vi "HFRR ADV v038.vi"() -> ()   [LabVIEW 2025] (continued)
                }
                n3063 = control-ref of="Tab Control 9"() -> (w3828:refnum<vi>)
                n3064 = call-dynamic "Append Control Image to Report.vi"("report in"=w3833, "alignment (default)"=HTML_Report_Image_Alignment."ABSMIDDLE", "ctrl reference"=w3828, "error in (no error)"=w3832) -> ("report out"=w3827:refnum<class "NI_report.lvclass">, "error out"=w3826:errorcluster)  [unwired: 8 in, 2 out]
                n3065 = for {
                  N: 3 -> [_]
                  tunnel: [w3860] -> w3811
                  tunnel: [w3859] -> w3810
                  tunnel: w3827 -> [w3858]
                  tunnel: w3826 -> [w3857]
                  n3066 = call-dynamic "New Report Line.vi"("report in"=w3858, "error in (no error)"=w3857) -> ("report out"=w3860:refnum<class "NI_report.lvclass">, "error out"=w3859:errorcluster)  [unwired: 12 in]
                }
                n3067 = for {
                  N: 100 -> [_]
                  tunnel: w3811 -> [w3856]
                  tunnel: w3810 -> [w3854]
                  tunnel: [w3855] -> w3807
                  tunnel: [w3853] -> w3805
                  n3068 = call-dynamic "Set Report Tab Width.vi"("report in"=w3856, "error in (no error)"=w3854) -> ("report out"=w3855:refnum<class "NI_report.lvclass">, "error out"=w3853:errorcluster)  [unwired: 12 in]
                }
                n3069 = String To Path(string="C:\\LAB-IQ\\im\\Temp_resized.jpg") -> (path=w3797:path)
                n3070 = call-poly <vilib>:"Append Image to Report.vi"("report in"=w3807, "path or URL of image"=w3797, "error in (no error)"=w3805) -> ("report out"=w3806:refnum<class "NI_report.lvclass">, "error out"=w3804:errorcluster)  [unwired: 9 in, 2 out]
                n3071 = call-poly <vilib>:"Open HTML Report in Browser.vi"("report in"=w3806, "error in (no error)"=w3804) -> ("report out"=w3841:refnum<class "NI_report.lvclass">, "error out"=w3840:errorcluster)  [unwired: 11 in, 1 out]
                n3072 = call-dynamic "Dispose Report.vi"("report in"=w3841, "error in (no error)"=w3840) -> ()  [unwired: 13 in, 1 out]
              }
              frame #2 {
              }
              frame #3 {
                n3073 = disable-structure shown="Disabled" {
                  frame Disabled {
                    n3074 = local read "String 10"() -> (w3881:string)
                    n3075 = Concatenate Strings("C:\\LAB-IQ-NXT\\Data\\" ("string"), w3881, ".jpg" ("string")) -> (w3879:string)
                    n3076 = String To Path(string=w3879) -> (path=w3878:path)
                    n3077 = Delete(path (use dialog)=w3878) -> ()  [unwired: 4 in, 3 out]
                  }
                  frame Enabled {
                  }
                }
                n3078 = local write "Print 2"(FALSE ("Print")) -> ()
              }
            }
          }
        }
      }
    }
    n3079 = Wait (ms)(milliseconds to wait=u32 50) -> ()  [unwired: 1 out]
    n3080 = Wait (ms)(milliseconds to wait=u32 50) -> ()  [unwired: 1 out]
    n3081 = local read "Quit"() -> (w2223:bool)
  }
  n3082 = VISA Close(VISA resource name=w41, error in (no error)=w40) -> ()  [unwired: 1 out]
  n3083 = while {
    stop <- w4032 stop-if-true
    n3084 = local read "Auto Start Test"() -> (w4030:bool)
    n3085 = local read "RUN"() -> (w4029:bool)
    n3086 = Wait (ms)(milliseconds to wait=u32 1000) -> ()  [unwired: 1 out]
    n3087 = Or(x=w4029, y=w4030) -> (x .or. y?=w4028:bool)
    n3088 = case shown="True" w4028 {
      frame False {
      }
      frame True {
        n3089 = local read "LVDT STROKE Actual"() -> (w4033:dbl)
        n3090 = In Range and Coerce(upper limit=1.2, x=w4033, lower limit=0.6) -> (In Range?=w4036:bool)  [unwired: 1 out]
        n3091 = call-poly <vilib>:"Random Number (Range).vi"("lower bound (0)"=0.998 ("upper bound (100)"), "upper bound (100)"=1.003) -> ("number"=w4034:dbl)  [unwired: 9 in]
        n3092 = case shown="True" w4036 {
          tunnel: [w4041 w4042] -> w4035
          tunnel: w4034 -> [_ w4042]
          tunnel: w4033 -> [w4041 _]
          frame False {
          }
          frame True {
          }
        }
        "LVDT STROKE DISPLAY" <- w4035
      }
    }
    n3093 = local read "Quit"() -> (w4032:bool)
  }
  n3094 = while {
    tunnel: [w4059] -> w49
    shift-right: [w4052] -> _
    shift-left: 0.0 -> [w4055]
    shift-right: [w4051] -> _
    shift-left: 0.0 -> [w4054]
    shift-right: [w4050] -> _
    shift-left: 100.0 ("vc_cmd") -> [w4053]
    stop <- w4059 stop-if-true
    # "PID LOGIC"
    n3095 = local read "run test Calibration"() -> (w4047:bool)
    n3096 = local read "RUN"() -> (w4057:bool)
    n3097 = local read "Auto Start Temp"() -> (w4048:bool)
    n3098 = local read "Auto Start Test"() -> (w4056:bool)
    n3099 = local read "START TEMP"() -> (w4046:bool)
    n3100 = And(x=w4048, y=w4056) -> (x .and. y?=w4049:bool)
    n3101 = Or(x=w4057, y=w4049) -> (x .or. y?=w4058:bool)
    n3102 = And(x=w4058, y=w4046) -> (x .and. y?=w4045:bool)
    n3103 = And(x=w4047, y=w4046) -> (x .and. y?=w4044:bool)
    n3104 = Or(x=w4044, y=w4045) -> (x .or. y?=w4043:bool)
    n3105 = Wait (ms)(milliseconds to wait="milliseconds to wait") -> ()  [unwired: 1 out]
    n3106 = case shown="True" w4043 {
      tunnel: [400.0 ("out_vc_cmd") w4078] -> w4050
      tunnel: [w4062 w4080] -> w4051
      tunnel: [w4062 w4079] -> w4052
      tunnel: w4055 -> [_ w4069]
      tunnel: w4054 -> [_ w4068]
      tunnel: w4053 -> [_ w4067]
      tunnel: w4047 -> [_ w4063]
      frame False {
        w4062 = 0.0 ("error_out")
      }
      frame True {
        n3107 = case shown="True" w4063 {
          tunnel: [w4087 1.0] -> w4065
          frame False {
            n3108 = local read "Set Strk"() -> (w4086:dbl)
            n3109 = Add(x=w4086, y="Add up Stroke") -> (x+y=w4087:dbl)
          }
          frame True {
          }
        }
        n3110 = local read "LVDT STROKE"() -> (w4064:dbl)
        n3111 = formula code="// Zero-Hardcode Explicit Positional-Form PID Engine\n// Inputs: target_stroke, measured_stroke, dt, prev_error, integral_accumulator_in, prev_vc_cmd\n//         kp, ki, kd, max_step_change, max_amplitude, min_amplitude, startup_cmd\n// Outputs: vc_cmd, error_out, out_error, integral_accumulator_out, out_vc_cmd\n\n// 1. Calculate Tracking Error\nfloat current_error = target_stroke - measured_stroke;\nerror_out = current_error;\n\n// 2. Compute Proportional Term\nfloat p_term = kp * current_error;\n\n// 3. Compute Derivative Term\nfloat d_term = 0.0;\nif (dt > 0.0) {\n    d_term = kd * ((current_error - prev_error) / dt);\n}\n\n// 4. Update and Accumulate Integral Term\nfloat current_integral = integral_accumulator_in + (current_error * dt);\nfloat i_term = ki * current_integral;\n\n// 5. Calculate Ideal Target Command (Anchored by startup baseline)\nfloat ideal_command = startup_cmd + p_term + i_term + d_term;\n\n// 6. Apply Loop Rate Limiting FIRST \n// (Forces the command to climb gradually from prev_vc_cmd instead of jumping straight to max)\nfloat raw_adjustment = ideal_command - prev_vc_cmd;\n\nif (raw_adjustment > max_step_change) {\n    raw_adjustment = max_step_change;\n} else if (raw_adjustment < -max_step_change) {\n    raw_adjustment = -max_step_change;\n}\n\nfloat next_vc_cmd = prev_vc_cmd + raw_adjustment;\n\n// 7. Anti-Windup Protection & Final Output Safety Safeguard Clamping\n// (Back-calculating based on what we are ACTUALLY outputting)\nif (next_vc_cmd > max_amplitude) {\n    float excess = next_vc_cmd - max_amplitude;\n    if (ki > 0.0) {\n        current_integral -= excess / ki;\n    }\n    next_vc_cmd = max_amplitude;\n} else if (next_vc_cmd < min_amplitude) {\n    float excess = next_vc_cmd - min_amplitude;\n    if (ki > 0.0) {\n        current_integral -= excess / ki;\n    }\n    next_vc_cmd = min_amplitude;\n}\n\n// 8. Map to Shift Registers for memory persistence\nvc_cmd = next_vc_cmd;\nout_error = current_error;                   \nintegral_accumulator_out = current_integral;  \nout_vc_cmd = next_vc_cmd;"("target_stroke"=w4065, "measured_stroke"=w4064, "dt"="dt", "integral_accumulator_in"=w4068, "prev_error"=w4069, "prev_vc_cmd"=w4067, "kp"="kp", "ki"="ki", "kd"="kd", "max_step_change"="max_step_change", "max_amplitude"="max_amplitude", "min_amplitude"="min_amplitude", "startup_cmd"="startup_cmd") -> ("vc_cmd"=w4084:dbl, "out_error"=w4079:dbl, "integral_accumulator_out"=w4080:dbl, "out_vc_cmd"=w4078:dbl)  [unwired: 1 out]
        "output Vpp" <- w4084
        n3112 = Number To Fractional String(number=w4084, precision (6)=i16 1) -> (F-format string=w4082:string)  [unwired: 2 in]
        n3113 = Concatenate Strings("DAC;" ("string"), w4082) -> (w4066:string)
        n3114 = local write "Due Write"(w4066) -> ()
        "prev_error" <- w4069
        "integral_accumulator_in" <- w4068
        "prev_vc_cmd" <- w4067
      }
    }
    n3115 = local read "Quit"() -> (w4059:bool)
  }
  n3116 = Or(x=w45, y=w44) -> (x .or. y?=w46:bool)
  n3117 = Or(x=w42, y=w46) -> (x .or. y?=w51:bool)
  n3118 = control-ref of="new picture"() -> ()  [unwired: 1 out]
  n3119 = Or(x=w54, y=w51) -> (x .or. y?=w48:bool)
  n3120 = Or(x=w48, y=w49) -> (x .or. y?=w43:bool)
  n3121 = while {
    tunnel: [w4089] -> w53
    i -> [w4096]
    stop <- w4089 stop-if-true
    n3122 = local read "Quit"() -> (w4089:bool)
    n3123 = Equal To 0?(x=w4096) -> (x = 0?=w4094:bool)
    n3124 = call "Elapsed Time3"("Time Target (s)"=45.0, "Auto Reset"=TRUE) -> ("Time has Elapsed"=w4093:bool)  [unwired: 10 in, 7 out]
    n3125 = Wait (ms)(milliseconds to wait=u32 50) -> ()  [unwired: 1 out]
    n3126 = Or(x=w4093, y=w4094) -> (x .or. y?=w4095:bool)
    n3127 = case shown="True" w4095 {
      frame False {
      }
      frame True {
        n3128 = call <vilib>:"System Exec.vi"("run minimized? (F)"=TRUE, "error in (no error)"="error in (no error)", "command line"="powercfg.exe -change -monitor-timeout-ac 0") -> ("error out"=w4107:errorcluster)  [unwired: 5 in, 3 out]
        n3129 = call <vilib>:"System Exec.vi"("run minimized? (F)"=TRUE, "error in (no error)"=w4107, "command line"="powercfg.exe -change -disk-timeout-ac 0") -> ("error out"=w4106:errorcluster)  [unwired: 5 in, 3 out]
        n3130 = call <vilib>:"System Exec.vi"("run minimized? (F)"=TRUE, "error in (no error)"=w4106, "command line"="powercfg.exe -change -standby-timeout-ac 0") -> ("error out"=w4105:errorcluster)  [unwired: 5 in, 3 out]
        n3131 = call <vilib>:"System Exec.vi"("run minimized? (F)"=TRUE, "error in (no error)"=w4105, "command line"="powercfg.exe -change -hibernate-timeout-ac 0") -> ("error out"=w4104:errorcluster)  [unwired: 5 in, 3 out]
        n3132 = call <vilib>:"Simple Error Handler.vi"("error in (no error)"=w4104) -> ("error out"=w4110:errorcluster)  [unwired: 4 in, 4 out]
        n3133 = call <vilib>:"Clear Errors.vi"("error in (no error)"=w4110) -> ("error out"=→"error out":errorcluster)  [unwired: 5 in, 1 out]
      }
    }
  }
  n3134 = Compound Arithmetic op=OR(w56, w43, w53) -> (w55:bool)
  n3135 = flat-sequence {
    tunnel: w55 -> [_]
    tunnel: [w4112] -> w25
    tunnel: w25 -> [_]
    frame #0 {
      n3136 = call "CLOSE CONNECTION.vi"() -> ("error out"=w4112:errorcluster)  [unwired: 11 in]
    }
    frame #1 {
      n3137 = Quit LabVIEW(quit? (T)=TRUE) -> ()
      n3138 = local write "Quit"(FALSE ("EXIT")) -> ()
    }
  }
  n3139 = property on="Heater Button" class="Bool (strict)"("Visible"=TRUE) -> ()  [unwired: 2 in, 2 out]
  n3140 = while {
    tunnel: [w4119] -> _
    i -> [w4119]
    stop <- w4115 stop-if-true
    # "Langauage selection"
    n3141 = Equal?(x="Lan flag", y=22.0) -> ()  [unwired: 1 out]
    n3142 = disable-structure shown="Disabled" {
      frame Disabled {
        n3143 = stacked-sequence {
          frame #0 {
            n3144 = case shown="\"Russian\"" "Language Selection" {
              tunnel: [0 1] -> w4121
              frame "English", Default {
              }
              frame "Russian" {
              }
            }
            n3145 = for {
              N: 130 -> [_]
              tunnel: "Table" -> [w4130]
              tunnel: w4121 -> [w4129]
              i -> [w4128]
              n3146 = Index Array(array=w4130, index (row)=w4128, index (col)=w4129) -> (element=w4127:string)
              n3147 = case shown="1" w4128 {
                tunnel: w4127 -> [w4131 w4132 _ w4133 w4134 w4135 w4136 w4137 w4138 w4139 w4140 w4141 w4142 w4143 w4144 w4145 w4146 w4147 w4148 w4149 w4150 w4151 w4152 w4153 w4154 w4155 w4156 w4157 w4158 _ _ w4159 w4160 w4161 w4162 w4163 w4164 w4173 w4180 w4187 w4194 w4198 w4201 w4204 w4206 w4208 w4209 w4210 w4211 w4212 w4213 w4214 w4215 w4216 w4217 w4218 w4219 w4220 w4221 w4222 w4223 w4224 w4225 w4226 w4227 w4228 w4229 w4230 w4231 w4232 w4233 w4234 w4235 w4236 w4237 w4238 w4239 w4240 w4241 w4242 w4243 w4244 w4245 w4246 w4247 w4248 w4249 w4250 w4251 w4252 w4253 w4254 w4255 w4256 w4257 w4258 w4259 w4260 w4261 w4262 w4263 w4264 w4265 w4266 w4267 _ w4268 w4269 w4270 w4271 w4272 w4273 w4274 w4275 w4276 w4277 w4278 w4279 w4280 _ w4281 w4282 w4283 w4284 w4285 w4286 _]
                frame 0 {
                  n3148 = local write "S"(w4131) -> ()
                }
                frame 1 {
                  n3149 = local write "S 2"(w4132) -> ()
                }
                frame 2 {
                }
                frame 3 {
                  n3150 = local write "S 4"(w4133) -> ()
                }
                frame 4 {
                  n3151 = property on="FILE" class="Str"("Caption.Text"=w4134) -> ()  [unwired: 2 in, 2 out]
                }
                frame 5 {
                  n3152 = property on="Fuel Discription :" class="Str"("Caption.Text"=w4135) -> ()  [unwired: 2 in, 2 out]
                }
                frame 6 {
                  n3153 = property on="Remarks :" class="Str"("Caption.Text"=w4136) -> ()  [unwired: 2 in, 2 out]
                }
                frame 7 {
                  n3154 = property on="Save & Continue" class="Bool (strict)"("Boolean Text.Text"=w4137) -> ()  [unwired: 2 in, 2 out]
                }
                frame 8 {
                }
                frame 9 {
                  n3155 = property on="Set Hz" class="DigNum (strict)"("Caption.Text"=w4139) -> ()  [unwired: 2 in, 2 out]
                }
                frame 10 {
                }
                frame 11 {
                  n3156 = property on="NORMAL LOAD" class="DigNum (strict)"("Caption.Text"=w4141) -> ()  [unwired: 2 in, 2 out]
                }
                frame 12 {
                }
                frame 13 {
                  n3157 = property on="Set Temp" class="DigNum (strict)"("Caption.Text"=w4143) -> ()  [unwired: 2 in, 2 out]
                }
                frame 14 {
                  n3158 = local write "S 15"(w4144) -> ()
                }
                frame 15 {
                  n3159 = property on="Set Rh" class="DigNum (strict)"("Caption.Text"=w4145) -> ()  [unwired: 2 in, 2 out]
                }
                frame 16 {
                }
                frame 17 {
                  n3160 = local write "S 18"(w4147) -> ()
                }
                frame 18 {
                  "String 17" <- w4148
                }
                frame 19 {
                  n3161 = property on="test time" class="DigNum (strict)"("Caption.Text"=w4149) -> ()  [unwired: 2 in, 2 out]
                }
                frame 20 {
                  "String 18" <- w4150
                  "String 22" <- w4150
                }
                frame 21 {
                  n3162 = property on="Elapsed time" class="DigNum (strict)"("Caption.Text"=w4151) -> ()  [unwired: 2 in, 2 out]
                }
                frame 22 {
                  n3163 = property on="Samplingtime 2" class="DigNum (strict)"("Caption.Text"=w4152) -> ()  [unwired: 2 in, 2 out]
                }
                frame 23 {
                  "String 21" <- w4153
                }
                frame 24 {
                  n3164 = property on="Countdown" class="DigNum (strict)"("Caption.Text"=w4154) -> ()  [unwired: 2 in, 2 out]
                }
                frame 25 {
                  n3165 = property on="Countdown 2" class="DigNum (strict)"("Caption.Text"=w4155) -> ()  [unwired: 2 in, 2 out]
                }
                frame 26 {
                  n3166 = property on="Engage" class="Bool (strict)"("Boolean Text.Text"=w4156) -> ()  [unwired: 2 in, 2 out]
                }
                frame 27 {
                  n3167 = property on="Boolean  4" class="Bool (strict)"("Boolean Text.Text"=w4157) -> ()  [unwired: 2 in, 2 out]
                }
                frame 28 {
                  n3168 = property on="Test \nStatus" class="Bool (strict)"("Boolean Text.Text"=w4158) -> ()  [unwired: 2 in, 2 out]
                }
                frame 29 {
                }
                frame 30 {
                }
                frame 31 {
                }
                frame 32 {
                  n3169 = property on="RSTCOF" class="Bool"("Boolean Text.Text"=w4160) -> ()  [unwired: 2 in, 2 out]
                  n3170 = property on="RST FF" class="Bool"("Boolean Text.Text"=w4160) -> ()  [unwired: 2 in, 2 out]
                  n3171 = property on="RST TEMP" class="Bool"("Boolean Text.Text"=w4160) -> ()  [unwired: 2 in, 2 out]
                  n3172 = property on="RSTV1 3" class="Bool"("Boolean Text.Text"=w4160) -> ()  [unwired: 2 in, 2 out]
                  n3173 = property on="rstv2" class="Bool"("Boolean Text.Text"=w4160) -> ()  [unwired: 2 in, 2 out]
                  n3174 = property on="RSTV1 2" class="Bool"("Boolean Text.Text"=w4160) -> ()  [unwired: 2 in, 2 out]
                  n3175 = property on="RST CP" class="Bool"("Boolean Text.Text"=w4160) -> ()  [unwired: 2 in, 2 out]
                }
                frame 33 {
                  "S 61" <- w4161
                }
                frame 34 {
                  "String 23" <- w4162
                }
                frame 35 {
                  n3176 = property on="Rh Before" class="DigNum (strict)"("Caption.Text"=w4163) -> ()  [unwired: 2 in, 2 out]
                }
                frame 36 {
                  n3177 = Match Pattern(string=w4164, regular expression=",") -> (before substring=→"bs":string, after substring=→"as":string)  [unwired: 1 in, 2 out]
                  n3178 = property on="Rh After" class="DigNum (strict)"("Caption.Text"=w4164) -> ()  [unwired: 2 in, 2 out]
                }
                frame 37 {
                  n3179 = Match Pattern(string=w4173, regular expression=",") -> (before substring=w4172:string, after substring=w4171:string)  [unwired: 1 in, 2 out]
                  "bs" <- w4172
                  "as" <- w4171
                  n3180 = Concatenate Strings(w4172, w4171) -> (w4168:string)
                  n3181 = property on="Humidity before test 2" class="DigNum (strict)"("Caption.Text"=w4168) -> ()  [unwired: 2 in, 2 out]
                  n3182 = Concatenate Strings(w4168, "=" ("string")) -> (w4169:string)
                  n3183 = local write "S 38"(w4169) -> ()
                }
                frame 38 {
                  n3184 = Match Pattern(string=w4180, regular expression=",") -> (before substring=w4179:string, after substring=w4178:string)  [unwired: 1 in, 2 out]
                  "bs" <- w4179
                  "as" <- w4178
                  n3185 = Concatenate Strings(w4179, w4178) -> (w4175:string)
                  n3186 = property on="Humidity after test 2" class="DigNum (strict)"("Caption.Text"=w4175) -> ()  [unwired: 2 in, 2 out]
                  n3187 = Concatenate Strings(w4175, "=" ("string")) -> (w4177:string)
                  n3188 = local write "S 39"(w4177) -> ()
                }
                frame 39 {
                  n3189 = Match Pattern(string=w4187, regular expression=",") -> (before substring=w4186:string, after substring=w4185:string)  [unwired: 1 in, 2 out]
                  "bs" <- w4186
                  "as" <- w4185
                  n3190 = Concatenate Strings(w4186, w4185) -> (w4182:string)
                  n3191 = property on="Temperature before test 2" class="DigNum (strict)"("Caption.Text"=w4182) -> ()  [unwired: 2 in, 2 out]
                  n3192 = Concatenate Strings(w4182, "=" ("string")) -> (→"String 34":string)
                }
                frame 40 {
                  n3193 = Match Pattern(string=w4194, regular expression=",") -> (before substring=w4193:string, after substring=w4192:string)  [unwired: 1 in, 2 out]
                  "bs" <- w4193
                  "as" <- w4192
                  n3194 = Concatenate Strings(w4193, w4192) -> (w4189:string)
                  n3195 = property on="Temperature after test 2" class="DigNum (strict)"("Caption.Text"=w4189) -> ()  [unwired: 2 in, 2 out]
                  n3196 = Concatenate Strings(w4189, "=" ("string")) -> (→"String 35":string)
                  n3197 = property on="Temperature after test" class="DigNum (strict)"("Caption.Text"=w4189) -> ()  [unwired: 2 in, 2 out]
                }
                frame 41 {
                  n3198 = property on="AVP 2" class="DigNum (strict)"("Caption.Text"=w4198) -> ()  [unwired: 2 in, 2 out]
                  n3199 = Concatenate Strings(w4198, "=" ("string")) -> (→"String 36":string)
                }
                frame 42 {
                  n3200 = property on="MWSD 2" class="DigNum (strict)"("Caption.Text"=w4201) -> ()  [unwired: 2 in, 2 out]
                  n3201 = Concatenate Strings(w4201, "=" ("string")) -> (→"String 37":string)
                }
                frame 43 {
                  n3202 = property on="HCF 2" class="DigNum (strict)"("Caption.Text"=w4204) -> ()  [unwired: 2 in, 2 out]
                  n3203 = Concatenate Strings(w4204, "=" ("string")) -> (→"String 38":string)
                }
                frame 44 {
                  n3204 = Concatenate Strings(w4206, "=" ("string")) -> (→"String 39":string)
                  n3205 = property on="WS1.4 2" class="DigNum (strict)"("Caption.Text"=w4206) -> ()  [unwired: 2 in, 2 out]
                }
                frame 45 {
                }
                frame 46 {
                  n3206 = local write "S 47"(w4209) -> ()
                }
                frame 47 {
                  n3207 = local write "S 48"(w4210) -> ()
                }
                frame 48 {
                  n3208 = local write "S 49"(w4211) -> ()
                }
                frame 49 {
                  n3209 = local write "S 50"(w4212) -> ()
                }
                frame 50 {
                  n3210 = local write "S 51"(w4213) -> ()
                }
                frame 51 {
                  n3211 = local write "S 52"(w4214) -> ()
                }
                frame 52 {
                  n3212 = local write "S 53"(w4215) -> ()
                }
                frame 53 {
                  n3213 = local write "S 54"(w4216) -> ()
                }
                frame 54 {
                  n3214 = local write "S 55"(w4217) -> ()
                }
                frame 55 {
                  n3215 = local write "S 56"(w4218) -> ()
                }
                frame 56 {
                  n3216 = local write "S 57"(w4219) -> ()
                }
                frame 57 {
                  n3217 = local write "S 58"(w4220) -> ()
                }
                frame 58 {
                  n3218 = local write "S 59"(w4221) -> ()
                }
                frame 59 {
                  n3219 = local write "S 60"(w4222) -> ()
                }
                frame 60 {
                  n3220 = local write "S 62"(w4223) -> ()
                }
                frame 61 {
                  n3221 = local write "S 63"(w4224) -> ()
                }
                frame 62 {
                  n3222 = local write "S 64"(w4225) -> ()
                }
                frame 63 {
                  n3223 = local write "S 65"(w4226) -> ()
                }
                frame 64 {
                  n3224 = local write "S 66"(w4227) -> ()
                }
                frame 65 {
                  n3225 = local write "S 67"(w4228) -> ()
                }
                frame 66 {
                  n3226 = local write "S 68"(w4229) -> ()
                }
                frame 67 {
                  n3227 = local write "S 69"(w4230) -> ()
                }
                frame 68 {
                  n3228 = local write "S 70"(w4231) -> ()
                }
                frame 69 {
                  n3229 = local write "S 71"(w4232) -> ()
                }
                frame 70 {
                  n3230 = local write "S 72"(w4233) -> ()
                }
                frame 71 {
                  n3231 = local write "S 73"(w4234) -> ()
                }
                frame 72 {
                  n3232 = local write "S 74"(w4235) -> ()
                }
                frame 73 {
                  n3233 = local write "S 75"(w4236) -> ()
                }
                frame 74 {
                  n3234 = local write "S 76"(w4237) -> ()
                }
                frame 75 {
                  n3235 = local write "S 77"(w4238) -> ()
                }
                frame 76 {
                  n3236 = local write "S 78"(w4239) -> ()
                }
                frame 77 {
                  n3237 = local write "S 79"(w4240) -> ()
                }
                frame 79 {
                  n3238 = property on="Sample Temperature ( °C )" class="XYGraph (strict)"("Y Scale.Name Label.Text"=w4241) -> ()  [unwired: 2 in, 2 out]
                }
                frame 80 {
                  n3239 = local write "S 81"(w4242) -> ()
                  n3240 = property on="Humidity ( %RH )" class="XYGraph (strict)"("Y Scale.Name Label.Text"=w4242) -> ()  [unwired: 2 in, 2 out]
                }
                frame 78 {
                  n3241 = property on="Air Temperature  ( °C )" class="XYGraph (strict)"("X Scale.Name Label.Text"=w4243) -> ()  [unwired: 2 in, 2 out]
                  n3242 = property on="Humidity ( %RH )" class="XYGraph (strict)"("X Scale.Name Label.Text"=w4243) -> ()  [unwired: 2 in, 2 out]
                  n3243 = property on="Sample Temperature ( °C )" class="XYGraph (strict)"("X Scale.Name Label.Text"=w4243) -> ()  [unwired: 2 in, 2 out]
                  n3244 = property on="Coefficient Of Friction" class="XYGraph (strict)"("X Scale.Name Label.Text"=w4243) -> ()  [unwired: 2 in, 2 out]
                }
                frame 81 {
                  n3245 = property on="Air Temperature  ( °C )" class="XYGraph (strict)"("Y Scale.Name Label.Text"=w4244) -> ()  [unwired: 2 in, 2 out]
                }
                frame 82 {
                  n3246 = local write "S 84"(w4245) -> ()
                }
                frame 83 {
                  n3247 = local write "S 85"(w4246) -> ()
                }
                frame 84 {
                  n3248 = local write "S 86"(w4247) -> ()
                }
                frame 85 {
                  n3249 = local write "S 87"(w4248) -> ()
                }
                frame 86 {
                  n3250 = local write "S 88"(w4249) -> ()
                }
                frame 87 {
                }
                frame 88 {
                  n3251 = local write "S 90"(w4251) -> ()
                }
                frame 89 {
                  n3252 = local write "S 91"(w4252) -> ()
                }
                frame 90 {
                  n3253 = local write "S 92"(w4253) -> ()
                }
                frame 91 {
                  n3254 = local write "S 93"(w4254) -> ()
                }
                frame 92 {
                  n3255 = local write "S 94"(w4255) -> ()
                }
                frame 93 {
                  n3256 = local write "S 95"(w4256) -> ()
                }
                frame 94 {
                  n3257 = local write "S 96"(w4257) -> ()
                }
                frame 95 {
                  n3258 = local write "S 97"(w4258) -> ()
                }
                frame 96 {
                  n3259 = local write "S 98"(w4259) -> ()
                }
                frame 97 {
                  n3260 = local write "S 99"(w4260) -> ()
                }
                frame 98 {
                  n3261 = local write "S 100"(w4261) -> ()
                }
                frame 99 {
                  n3262 = local write "S 101"(w4262) -> ()
                }
                frame 100 {
                  n3263 = local write "S 102"(w4263) -> ()
                }
                frame 101 {
                  n3264 = local write "S 103"(w4264) -> ()
                }
                frame 102 {
                  n3265 = local write "S 104"(w4265) -> ()
                }
                frame 103 {
                  n3266 = local write "S 105"(w4266) -> ()
                }
                frame 104 {
                  n3267 = local write "S 106"(w4267) -> ()
                }
                frame 105 {
                }
                frame 106 {
                  n3268 = property on="OK Button 17" class="Bool (strict)"("Boolean Text.Text"=w4268) -> ()  [unwired: 2 in, 2 out]
                }
                frame 107 {
                  n3269 = property on="OK Button 16" class="Bool (strict)"("Boolean Text.Text"=w4269) -> ()  [unwired: 2 in, 2 out]
                }
                frame 108 {
                  n3270 = property on="TITTLE" class="Str"("Caption.Text"=w4270) -> ()  [unwired: 2 in, 2 out]
                }
                frame 109 {
                  "String 30" <- w4271
                }
                frame 110 {
                  n3271 = property on="Test Date" class="Str"("Caption.Text"=w4272) -> ()  [unwired: 2 in, 2 out]
                  "String 31" <- w4272
                }
                frame 111 {
                  n3272 = property on="Sample ID" class="Str"("Caption.Text"=w4273) -> ()  [unwired: 2 in, 2 out]
                  "String 32" <- w4273
                }
                frame 112 {
                  n3273 = property on="Tested by" class="Str"("Caption.Text"=w4274) -> ()  [unwired: 2 in, 2 out]
                  "String 33" <- w4274
                }
                frame 113 {
                  n3274 = property on="System Configured Printers 2" class="Arr (strict)"("Caption.Text"=w4275) -> ()  [unwired: 2 in, 2 out]
                }
                frame 114 {
                  n3275 = property on="Selected Printer" class="Str"("Caption.Text"=w4276) -> ()  [unwired: 2 in, 2 out]
                }
                frame 115 {
                  n3276 = property on="Select Printer 3" class="DigNum (strict)"("Caption.Text"=w4277) -> ()  [unwired: 2 in, 2 out]
                }
                frame 116 {
                  n3277 = property on="Print" class="Bool (strict)"("Boolean Text.Text"=w4278) -> ()  [unwired: 2 in, 2 out]
                }
                frame 117 {
                  "String 41" <- w4279
                }
                frame 118 {
                  n3278 = property on="tested by" class="Str"("Caption.Text"=w4280) -> ()  [unwired: 2 in, 2 out]
                }
                frame 119 {
                }
                frame 120 {
                  n3279 = property on="Export" class="Bool (strict)"("Boolean Text.Text"=w4281) -> ()  [unwired: 2 in, 2 out]
                }
                frame 121 {
                }
                frame 122 {
                }
                frame 123 {
                  n3280 = property on="Select File Type" class="Enum (strict)"("Caption.Text"=w4284) -> ()  [unwired: 2 in, 2 out]
                }
                frame 124 {
                  n3281 = property on="s.NO" class="Str"("Caption.Text"=w4285) -> ()  [unwired: 2 in, 2 out]
                  "String 45" <- w4285
                }
                frame 125 {
                  n3282 = property on="trip1 8" class="Bool (strict)"("Boolean Text.Text"=w4286) -> ()  [unwired: 2 in, 2 out]
                }
                frame 126, Default {
                }
              }
            }
          }
          frame #1 {
            w4294 = TRUE ("Visible")
            n3283 = local read "S 91"() -> (w4311:string)
            n3284 = local read "S 90"() -> (w4310:string)
            n3285 = local read "S 88"() -> (w4309:string)
            n3286 = property on="File Path" class="Path"("Caption.Text"=w4310) -> ()  [unwired: 2 in, 2 out]
            n3287 = local read "S 71"() -> (w4304:string)
            n3288 = local read "S 86"() -> (w4306:string)
            n3289 = local read "S 85"() -> (w4307:string)
            n3290 = local read "S 87"() -> (w4305:string)
            n3291 = local read "S 84"() -> (w4308:string)
            n3292 = local read "S 103"() -> (w4293:string)
            n3293 = local read "S 104"() -> (w4292:string)
            n3294 = property on="Password" class="Str"("Caption.Text"=w4307) -> ()  [unwired: 2 in, 2 out]
            n3295 = property on="EDIT" class="Bool (strict)"("Boolean Text.Text"=w4304) -> ()  [unwired: 2 in, 2 out]
            n3296 = property on="SAVE" class="Bool (strict)"("Boolean Text.Text"=w4308) -> ()  [unwired: 2 in, 2 out]
            n3297 = Build Array(w4293, w4292) -> (w4291:string[])
            n3298 = property on="Heater Button" class="Bool (strict)"("Strings [4]"=w4291) -> ()  [unwired: 2 in, 2 out]
            n3299 = local read "S 92"() -> (w4303:string)
            n3300 = local read "S 93"() -> (w4302:string)
            n3301 = local read "S 105"() -> (w4289:string)
            n3302 = local read "S 106"() -> (w4288:string)
            n3303 = Build Array(w4303, w4302) -> ()  [unwired: 1 out]
            n3304 = Build Array(w4289, w4288) -> (w4290:string[])
            n3305 = local read "S 95"() -> (w4300:string)
            n3306 = local read "S 94"() -> (w4301:string)
            n3307 = local read "bs"() -> (w4316:string)
            n3308 = local read "as"() -> (w4317:string)
            n3309 = property on="Humidity" class="Bool (strict)"("Strings [4]"=w4290) -> ()  [unwired: 2 in, 2 out]
            n3310 = Concatenate Strings(w4316, "\r", w4317) -> ()  [unwired: 1 out]
            n3311 = property on="Rh After" class="DigNum (strict)"("Caption.Size to Text?"=TRUE ("Caption.Size to Text")) -> ()  [unwired: 2 in, 2 out]
            n3312 = local read "S 48"() -> (w4340:string)
            n3313 = local read "S 50"() -> (w4338:string)
            n3314 = local read "S 51"() -> (w4337:string)
            n3315 = local read "S 49"() -> (w4339:string)
            n3316 = local read "S 52"() -> (w4336:string)
            n3317 = local read "as"() -> (w4321:string)
            n3318 = local read "bs"() -> (w4322:string)
            n3319 = local read "S 56"() -> (w4335:string)
            n3320 = local read "S 57"() -> (w4334:string)
            n3321 = local read "S 58"() -> (w4333:string)
            n3322 = local read "S 59"() -> (w4332:string)
            n3323 = property on="OPEN" class="Bool (strict)"("Boolean Text.Text"=w4336) -> ()  [unwired: 2 in, 2 out]
            n3324 = property on="OPEN 1" class="Bool (strict)"("Boolean Text.Text"=w4340) -> ()  [unwired: 2 in, 2 out]
            n3325 = property on="OPEN 2" class="Bool (strict)"("Boolean Text.Text"=w4339) -> ()  [unwired: 2 in, 2 out]
            n3326 = property on="OPEN 3" class="Bool (strict)"("Boolean Text.Text"=w4338) -> ()  [unwired: 2 in, 2 out]
            n3327 = property on="OPEN 4" class="Bool (strict)"("Boolean Text.Text"=w4337) -> ()  [unwired: 2 in, 2 out]
            n3328 = Concatenate Strings(w4322, "\r", w4321) -> ()  [unwired: 1 out]
            n3329 = local read "S 102"() -> (w4295:string)
            n3330 = property on="КОФ1" class="DigNum (strict)"("Caption.Text"=w4335) -> ()  [unwired: 2 in, 2 out]
            n3331 = local read "S 98"() -> (w4299:string)
            n3332 = local read "S 99"() -> (w4298:string)
            n3333 = local read "S 100"() -> (w4297:string)
            n3334 = local read "S 101"() -> (w4296:string)
            n3335 = property on="КОФ2" class="DigNum (strict)"("Caption.Text"=w4334) -> ()  [unwired: 2 in, 2 out]
            n3336 = property on="КОФ3" class="DigNum (strict)"("Caption.Text"=w4333) -> ()  [unwired: 2 in, 2 out]
            n3337 = property on="КОФ4" class="DigNum (strict)"("Caption.Text"=w4332) -> ()  [unwired: 2 in, 2 out]
            n3338 = local read "bs"() -> (w4320:string)
            n3339 = local read "as"() -> (w4319:string)
            n3340 = local read "S 60"() -> (w4331:string)
            n3341 = local read "S 54"() -> (w4341:string)
            n3342 = Concatenate Strings(w4320, "\r", w4319) -> ()  [unwired: 1 out]
            n3343 = Concatenate Strings(w4341, w4331) -> ()  [unwired: 1 out]
            n3344 = local read "S 77"() -> (→"String 43":string)
            n3345 = local read "S 76"() -> (w4314:string)
            n3346 = local read "S 78"() -> (w4313:string)
            n3347 = local read "S 71"() -> (w4325:string)
            n3348 = local read "S 66"() -> (w4330:string)
            n3349 = local read "S 67"() -> (w4329:string)
            n3350 = local read "S 68"() -> (w4328:string)
            n3351 = local read "S 69"() -> (w4327:string)
            n3352 = local read "S 70"() -> (w4326:string)
            n3353 = property on="AIR TEMP" class="DigNum (strict)"("Caption.Text"=w4313) -> ()  [unwired: 2 in, 2 out]
            n3354 = property on="Set Strk" class="DigNum (strict)"("Caption.Text"=w4314) -> ()  [unwired: 2 in, 2 out]
            n3355 = property on="SPEED OUT:" class="DigNum (strict)"("Caption.Text"=w4328) -> ()  [unwired: 2 in, 2 out]
            n3356 = property on="EDIT" class="Bool (strict)"("Boolean Text.Text"=w4325) -> ()  [unwired: 2 in, 2 out]
            n3357 = local read "S 79"() -> (w4312:string)
          }
          frame #2 {
          }
        }
        n3358 = local write "Lan flag"(10.0 ("Lan flag")) -> ()
      }
      frame Enabled {
      }
    }
    n3359 = Wait (ms)(milliseconds to wait=u32 2000) -> ()  [unwired: 1 out]
    n3360 = local read "Quit"() -> (w4115:bool)
  }
  n3361 = while {
    shift-right: [w4347] -> _
    shift-left: _ -> [w4348]
    shift-right: [w4345] -> _
    shift-left: T18 {"Read Heave and Surge"="", "Bytes at Heave Port"=0.0, "Heave and Surge COM Port:"="COM9", "Com Port 2"="COM7", "Residual Due"="", "Heave COM Status 2"=TRUE, "Heave COM Status"=TRUE, "Port 2"=TRUE, "Sway PPR"=6400.0, "Surge PPR"=6400.0, "Heave PPR"=6400.0, "Sway Pitch"=2.0, "Surge Pitch"=3.0, "Heave Pitch"=4.0, "Sway Pulses/mm"=320.0, "Surge Pulses/mm"=1600.0, "Heave Pulses/mm"=1600.0, "inner loop"=0.0, "Read Heave and Surge 2"="", "String 36"="", "Write S"=FALSE, "WriteCC1"=[""], "Heave COM Loop"=0, "LastCom"="", "EXIT"=FALSE, "Error Heave"={"status"=TRUE, "code"=-1073807343, "source"=""}} -> [w4344]
    shift-right: [w4342] -> _
    shift-left: enum16{"init", "MAIN", "Panel Close"}."init" -> [w4343]
    stop <- w4346 stop-if-true
    # "HUMIDITY LOOP LOGIC"
    n3362 = case shown="\"MAIN\"" w4343 {
      tunnel: w4348 -> [w4362 w4386 w4450 w4452]
      tunnel: [w4357 w4373 w4450 w4452] -> w4347
      tunnel: [_ _ TRUE _] -> w4346
      tunnel: [w4354 w4371 w4448 w4451] -> w4345
      tunnel: w4344 -> [w4359 w4385 w4448 w4451]
      tunnel: [enum16{"init", "MAIN", "Panel Close"}."MAIN" w4380 _ _] -> w4342
      frame "init" {
        n3363 = local read "C3 :"() -> (w4349:refnum<visa-resource-name>)
        n3364 = Bundle By Name(cluster=w4359, "Heave and Surge COM Port:"=w4349) -> (w4358:T18)
        n3365 = call "Instrument fgv uno.vi"("Enum"=T32."INIT", "error in (no error) 2"=w4362, "INPUT"=w4358) -> ("error"=w4360:errorcluster, "output"=w4356:T18)  [unwired: 6 in, 1 out]
        n3366 = case shown="Error" w4360 {
          selector: w4360 -> [w4364 _]
          tunnel: [w4364 w4368] -> w4357
          tunnel: w4356 -> [w4363 w4366]
          tunnel: [w4363 w4365] -> w4355
          frame No Error {
          }
          frame Error {
            n3367 = call "Instrument fgv uno.vi"("Enum"=T32."ERROR INIT", "INPUT"=w4366) -> ("error"=w4369:errorcluster, "output"=w4365:T18)  [unwired: 7 in, 1 out]
            n3368 = call <vilib>:"Clear Errors.vi"("error in (no error)"=w4369) -> ("error out"=w4368:errorcluster)  [unwired: 5 in, 1 out]
          }
        }
        n3369 = local read "LastCom Humidity"() -> (w4352:string)
        n3370 = Unbundle By Name(w4355) -> ("Heave COM Status 2"=→"COM Status":bool, "Error Heave"=→"Error":errorcluster)  [unwired: 1 out]
        n3371 = Bundle By Name(cluster=w4355, "LastCom"=w4352) -> (w4354:T18)
      }
      frame "MAIN" {
        n3372 = Unbundle By Name(w4385) -> ("Com Port 2"=w4375:refnum<visa-resource-name>)
        n3373 = local read "C3 :"() -> (w4376:refnum<visa-resource-name>)
        n3374 = local write "COM Port Humidity :"(w4375) -> ()
        n3375 = Bundle By Name(cluster=w4385, "Heave and Surge COM Port:"=w4376) -> (w4384:T18)
        n3376 = Equal?(x=w4375, y=w4376) -> (x = y?=w4389:bool)
        n3377 = case shown="True" w4389 {
          tunnel: [w4404 w4421] -> w4374
          tunnel: w4386 -> [w4405 w4427]
          tunnel: w4384 -> [w4403 w4425]
          tunnel: [w4402 w4420] -> w4372
          frame False {
            n3378 = call <vilib>:"Clear Errors.vi"("error in (no error)"=w4405) -> ("error out"=w4401:errorcluster)  [unwired: 5 in, 1 out]
            n3379 = call "Instrument fgv uno.vi"("Enum"=T32."ERROR INIT", "error in (no error) 2"=w4401, "INPUT"=w4403) -> ("error"=w4407:errorcluster, "output"=w4402:T18)  [unwired: 6 in, 1 out]
            n3380 = call <vilib>:"Clear Errors.vi"("error in (no error)"=w4407) -> ("error out"=w4404:errorcluster)  [unwired: 5 in, 1 out]
          }
          frame True {
            n3381 = call "Instrument fgv uno.vi"("Enum"=T32."READ", "error in (no error) 2"=w4427, "INPUT"=w4425) -> ("error"=w4426:errorcluster, "output"=w4419:T18)  [unwired: 6 in, 1 out]
            n3382 = Bundle By Name(cluster=w4419, "String 36"="WRITE HUMIDITY") -> (w4418:T18)
            n3383 = case shown="True" "Write Humidity" {
              selector: "Write Humidity" -> [_ w4447]
              tunnel: w4426 -> [w4440 w4446]
              tunnel: [w4440 w4445] -> w4416
              tunnel: w4418 -> [w4439 w4443]
              tunnel: [w4439 w4442] -> w4415
              frame False {
              }
              frame True {
                n3384 = Not(x=w4447) -> (.not. x?=w4441:bool)
                n3385 = local write "Write Humidity"(w4441) -> ()
                n3386 = call "Instrument fgv uno.vi"("Enum"=T32."MANUAL WRITE", "error in (no error) 2"=w4446, "INPUT"=w4443) -> ("error"=w4445:errorcluster, "output"=w4442:T18)  [unwired: 6 in, 1 out]
              }
            }
            n3387 = Array Size(array="WriteHumidity") -> (size(s)=w4413:i32)
            n3388 = Greater Than 0?(x=w4413) -> (x > 0?=w4412:bool)
            n3389 = call "Instrument fgv uno.vi"("Enum"=T32."WRITE", "error in (no error) 2"=w4416, "WriteCC1"="WriteHumidity", "INPUT"=w4415) -> ("error"=w4423:errorcluster, "WriteCC1 2"=w4414:string[], "output"=w4422:T18)  [unwired: 5 in]
            n3390 = case shown="True" w4412 {
              tunnel: w4414 -> [_ w4429]
              frame False {
              }
              frame True {
                n3391 = local write "WriteHumidity"(w4429) -> ()
              }
            }
            n3392 = case shown="No Error" w4423 {
              selector: w4423 -> [w4430 w4433]
              tunnel: w4422 -> [w4431 w4438]
              tunnel: [w4431 w4437] -> w4420
              tunnel: [w4430 w4435] -> w4421
              frame No Error {
              }
              frame Error {
                n3393 = call <vilib>:"Clear Errors.vi"("error in (no error)"=w4433) -> ("error out"=w4432:errorcluster)  [unwired: 5 in, 1 out]
                n3394 = call "Instrument fgv uno.vi"("Enum"=T32."ERROR INIT", "error in (no error) 2"=w4432, "INPUT"=w4438) -> ("error"=w4436:errorcluster, "output"=w4437:T18)  [unwired: 6 in, 1 out]
                n3395 = call <vilib>:"Clear Errors.vi"("error in (no error)"=w4436) -> ("error out"=w4435:errorcluster)  [unwired: 5 in, 1 out]
              }
            }
            n3396 = Unbundle By Name(w4420) -> ("LastCom"=→"LastCom Humidity":string, "Read Heave and Surge"=→"Read HUMIDITY":string)
          }
        }
        n3397 = Unbundle By Name(w4372) -> ("Heave COM Status 2"=w4388:bool, "Error Heave"=w4377:errorcluster, "Bytes at Heave Port"=→"Bytes at Humidity Port  2":dbl)  [unwired: 1 out]
        n3398 = Unbundle By Name(w4377) -> ("status"=→"Humidity Port":bool)
        n3399 = Not(x=w4388) -> (.not. x?=w4378:bool)
        n3400 = local write "Error"(w4377) -> ()
        n3401 = local read "Quit"() -> (w4381:bool)
        n3402 = local write "COM Status"(w4378) -> ()
        n3403 = Select(t=enum16{"init", "MAIN", "Panel Close"}."Panel Close", s=w4381, f=enum16{"init", "MAIN", "Panel Close"}."MAIN") -> (s? t:f=w4380:enum16{"init", "MAIN", "Panel Close"})
        n3404 = local read "Humidity"() -> (w4370:bool)
        n3405 = case shown="True" w4370 {
          selector: w4370 -> [_ w4392]
          tunnel: w4374 -> [w4390 w4397]
          tunnel: [w4390 w4396] -> w4373
          tunnel: w4372 -> [w4391 w4395]
          tunnel: [w4391 w4394] -> w4371
          frame False {
          }
          frame True {
            n3406 = Not(x=w4392) -> (.not. x?=→"Humidity":bool)
            n3407 = call <vilib>:"Clear Errors.vi"("error in (no error)"=w4397) -> ("error out"=w4400:errorcluster)  [unwired: 5 in, 1 out]
            n3408 = call "Instrument fgv uno.vi"("Enum"=T32."ERROR INIT", "error in (no error) 2"=w4400, "INPUT"=w4395) -> ("error"=w4398:errorcluster, "output"=w4394:T18)  [unwired: 6 in, 1 out]
            n3409 = call <vilib>:"Clear Errors.vi"("error in (no error)"=w4398) -> ("error out"=w4396:errorcluster)  [unwired: 5 in, 1 out]
          }
        }
      }
      frame "Panel Close" {
      }
      frame Default {
      }
    }
  }
  n3410 = while {
    stop <- w4454 stop-if-true
    n3411 = call <vilib>:"High Resolution Polling Wait.vi"("seconds to wait"=0.05) -> ()  [unwired: 10 in, 1 out]
    n3412 = disable-structure shown="Enabled" {
      frame Disabled {
        n3413 = local read "Read HUMIDITY"() -> (w4455:string)
        n3414 = Spreadsheet String To Array(delimiter (Tab)=",", format string="", spreadsheet string=w4455, array type (2D Dbl)=string[] []) -> (array=w4474:string[])
        n3415 = for {
          tunnel: w4474 -> [w4483] mode=indexing
          tunnel: string[] ["STATE;", "SET;", "RH;", "T;", "AMB_RH;", "AMB_T;", "PUMP;", "FAN_IN;", "FAN_OUT;", "DEHUM;", "CURRENT;", "STALL;"] -> [w4482] mode=indexing
          tunnel: [w4481] -> w4473 mode=indexing
          n3416 = Match Pattern(string=w4483, regular expression=w4482) -> (after substring=w4481:string)  [unwired: 1 in, 3 out]
        }
        n3417 = Index Array(array=w4473) -> (element #1=→"STATE :":string, element #2=→"SET :":string, element #3=w4463:string, element #4=→"T :":string, element #5=w4461:string, element #6=→"AMB_T :":string, element #7=→"PUMP :":string, element #8=→"FAN_IN :":string, element #9=→"FAN_OUT :":string, element #10=→"DEHUM :":string, element #11=→"CURRENT :":string, element #12=→"STALL :":string)  [unwired: 12 in]
        "RH :" <- w4463
        "AMB_RH :" <- w4461
        n3418 = Fract/Exp String To Number(string=w4463) -> (number=w4456:dbl)  [unwired: 3 in, 1 out]
        n3419 = Fract/Exp String To Number(string=w4461) -> (number=w4460:dbl)  [unwired: 3 in, 1 out]
        n3420 = local write "Ambient Humidity :"(w4460) -> ()
        n3421 = Equal?(x=w4456, y=0.0) -> (x = y?=w4458:bool)
        n3422 = case shown="True" w4458 {
          tunnel: [w4479 w4480] -> w4457
          tunnel: w4456 -> [w4479 _]
          frame False {
            (unwired) 0.0
            "Humidity temp" <- w4479
          }
          frame True {
            n3423 = local read "Humidity temp"() -> (w4480:dbl)
          }
        }
        "RH Numeric:" <- w4457
      }
      frame Enabled {
        n3424 = local read "Read HUMIDITY"() -> (w4503:string)
        n3425 = Spreadsheet String To Array(delimiter (Tab)=",", format string="", spreadsheet string=w4503, array type (2D Dbl)=dbl[] []) -> (array=w4499:dbl[])
        n3426 = Index Array(array=w4499) -> (element #1=→"STATE :":dbl, element #2=→"SET :":dbl, element #3=w4484:dbl, element #4=→"T :":dbl, element #5=→"AMB_RH :":dbl, element #6=→"AMB_T :":dbl, element #7=→"PUMP :":dbl, element #8=→"FAN_IN :":dbl, element #9=→"FAN_OUT :":dbl, element #10=→"DEHUM :":dbl, element #11=→"CURRENT :":dbl, element #12=→"STALL":dbl)  [unwired: 12 in]
        "RH :" <- w4484
        n3427 = Equal?(x=w4484, y=0.0) -> (x = y?=w4487:bool)
        n3428 = case shown="False" w4487 {
          tunnel: [w4504 w4505] -> w4488
          tunnel: w4484 -> [w4504 _]
          frame False {
            "Humidity temp 2" <- w4504
          }
          frame True {
            n3429 = local read "Humidity temp 2"() -> (w4505:dbl)
          }
        }
        n3430 = local write "RH Numeric:"(w4488) -> ()
      }
    }
    n3431 = local read "Quit"() -> (w4454:bool)
  }
  n3432 = while {
    shift-right: [w4511] -> _
    shift-left: _ -> [w4512]
    shift-right: [w4509] -> _
    shift-left: T20 {"Read Uno"="", "Bytes at Heave Port"=0.0, "UNO COM Port:"="COM9", "UNO COM Port: 2"="COM7", "Residual Due"="", "UNO COM Status 2"=TRUE, "UNO COM Status"=TRUE, "Port 2"=TRUE, "Sway PPR"=6400.0, "Surge PPR"=6400.0, "Heave PPR"=6400.0, "Sway Pitch"=2.0, "Surge Pitch"=3.0, "Heave Pitch"=4.0, "Sway Pulses/mm"=320.0, "Surge Pulses/mm"=1600.0, "Heave Pulses/mm"=1600.0, "inner loop"=0.0, "Read Heave and Surge 2"="", "String 36"="", "Write S"=FALSE, "WriteCC1"=[""], "Heave COM Loop"=0, "LastCom"="", "EXIT"=FALSE, "Error Heave"={"status"=TRUE, "code"=-1073807343, "source"=""}} -> [w4508]
    shift-right: [w4506] -> _
    shift-left: enum16{"init", "MAIN", "Panel Close"}."init" -> [w4507]
    stop <- w4510 stop-if-true
    # "UNO CODE LOGIC"
    n3433 = case shown="\"MAIN\"" w4507 {
      tunnel: w4512 -> [w4526 w4545 w4601 w4603]
      tunnel: [w4521 w4550 w4601 w4603] -> w4511
      tunnel: [_ _ TRUE _] -> w4510
      tunnel: [w4517 w4548 w4599 w4602] -> w4509
      tunnel: w4508 -> [w4523 w4544 w4599 w4602]
      tunnel: [enum16{"init", "MAIN", "Panel Close"}."MAIN" w4539 _ _] -> w4506
      frame "init" {
        n3434 = local read "Com Port 1"() -> (w4513:refnum<visa-resource-name>)
        n3435 = Bundle By Name(cluster=w4523, "UNO COM Port:"=w4513) -> (w4522:T20)
        n3436 = call "Instrument fgv.vi"("Enum"=T32."INIT", "error in (no error) 2"=w4526, "INPUT"=w4522) -> ("error"=w4524:errorcluster, "output"=w4520:T18)  [unwired: 6 in, 1 out]
        n3437 = case shown="Error" w4524 {
          selector: w4524 -> [w4528 _]
          tunnel: [w4528 w4532] -> w4521
          tunnel: w4520 -> [w4527 w4530]
          tunnel: [w4527 w4529] -> w4518
          frame No Error {
          }
          frame Error {
            n3438 = call "Instrument fgv.vi"("Enum"=T32."ERROR INIT", "INPUT"=w4530) -> ("error"=w4533:errorcluster, "output"=w4529:T18)  [unwired: 7 in, 1 out]
            n3439 = call <vilib>:"Clear Errors.vi"("error in (no error)"=w4533) -> ("error out"=w4532:errorcluster)  [unwired: 5 in, 1 out]
          }
        }
        n3440 = local read "LastCom UNO"() -> (w4515:string)
        n3441 = Unbundle By Name(w4518) -> ("Heave COM Status 2"=→"Instrument Status":bool, "Error Heave"=→"Error  2":errorcluster)  [unwired: 1 out]
        n3442 = Bundle By Name(cluster=w4518, "LastCom"=w4515) -> (w4517:T18)
      }
      frame "MAIN" {
        n3443 = Unbundle By Name(w4544) -> ("UNO COM Port: 2"=w4534:refnum<visa-resource-name>)
        n3444 = local read "Com Port 1"() -> (w4535:refnum<visa-resource-name>)
        n3445 = local write "COM Port UNO :"(w4534) -> ()
        n3446 = Equal?(x=w4534, y=w4535) -> (x = y?=w4551:bool)
        n3447 = Bundle By Name(cluster=w4544, "UNO COM Port:"=w4535) -> (w4543:T20)
        n3448 = case shown="True" w4551 {
          tunnel: [w4555 w4572] -> w4550
          tunnel: w4545 -> [w4556 w4578]
          tunnel: w4543 -> [w4554 w4576]
          tunnel: [w4553 w4571] -> w4548
          frame False {
            n3449 = call <vilib>:"Clear Errors.vi"("error in (no error)"=w4556) -> ("error out"=w4552:errorcluster)  [unwired: 5 in, 1 out]
            n3450 = call "Instrument fgv.vi"("Enum"=T32."ERROR INIT", "error in (no error) 2"=w4552, "INPUT"=w4554) -> ("error"=w4558:errorcluster, "output"=w4553:T18)  [unwired: 6 in, 1 out]
            n3451 = call <vilib>:"Clear Errors.vi"("error in (no error)"=w4558) -> ("error out"=w4555:errorcluster)  [unwired: 5 in, 1 out]
          }
          frame True {
            n3452 = call "Instrument fgv.vi"("Enum"=T32."READ", "error in (no error) 2"=w4578, "INPUT"=w4576) -> ("error"=w4577:errorcluster, "output"=w4570:T18)  [unwired: 6 in, 1 out]
            n3453 = Bundle By Name(cluster=w4570, "String 36"="WRITE UNO") -> (w4569:T18)
            n3454 = case shown="True" "Write" {
              selector: "Write" -> [_ w4593]
              tunnel: w4577 -> [w4591 w4598]
              tunnel: [w4591 w4597] -> w4567
              tunnel: w4569 -> [w4590 w4595]
              tunnel: [w4590 w4594] -> w4566
              frame False {
              }
              frame True {
                n3455 = Not(x=w4593) -> (.not. x?=w4592:bool)
                n3456 = local write "Write"(w4592) -> ()
                n3457 = call "Instrument fgv.vi"("Enum"=T32."MANUAL WRITE", "error in (no error) 2"=w4598, "INPUT"=w4595) -> ("error"=w4597:errorcluster, "output"=w4594:T18)  [unwired: 6 in, 1 out]
              }
            }
            n3458 = Array Size(array="Write UNO") -> (size(s)=w4564:i32)
            n3459 = Greater Than 0?(x=w4564) -> (x > 0?=w4563:bool)
            n3460 = call "Instrument fgv.vi"("Enum"=T32."WRITE", "error in (no error) 2"=w4567, "WriteCC1"="Write UNO", "INPUT"=w4566) -> ("error"=w4574:errorcluster, "WriteCC1 2"=w4565:string[], "output"=w4573:T18)  [unwired: 5 in]
            n3461 = case shown="True" w4563 {
              tunnel: w4565 -> [_ w4580]
              frame False {
              }
              frame True {
                n3462 = local write "Write UNO"(w4580) -> ()
              }
            }
            n3463 = case shown="Error" w4574 {
              selector: w4574 -> [w4581 w4584]
              tunnel: w4573 -> [w4582 w4589]
              tunnel: [w4582 w4588] -> w4571
              tunnel: [w4581 w4586] -> w4572
              frame No Error {
              }
              frame Error {
                n3464 = call <vilib>:"Clear Errors.vi"("error in (no error)"=w4584) -> ("error out"=w4583:errorcluster)  [unwired: 5 in, 1 out]
                n3465 = call "Instrument fgv.vi"("Enum"=T32."ERROR INIT", "error in (no error) 2"=w4583, "INPUT"=w4589) -> ("error"=w4587:errorcluster, "output"=w4588:T18)  [unwired: 6 in, 1 out]
                n3466 = call <vilib>:"Clear Errors.vi"("error in (no error)"=w4587) -> ("error out"=w4586:errorcluster)  [unwired: 5 in, 1 out]
              }
            }
            n3467 = Unbundle By Name(w4571) -> ("LastCom"=→"LastCom UNO":string, "Read Heave and Surge"=→"Read UNO":string)
          }
        }
        n3468 = Unbundle By Name(w4548) -> ("Heave COM Status 2"=w4549:bool, "Heave COM Status"=w4538:bool, "Error Heave"=w4536:errorcluster, "Bytes at Heave Port"=→"Bytes at Humidity Port":dbl)
        n3469 = Not(x=w4538) -> (.not. x?=w4546:bool)
        n3470 = Not(x=w4549) -> (.not. x?=w4537:bool)
        n3471 = local write "Instrument Status"(w4546) -> ()
        n3472 = local write "Error  2"(w4536) -> ()
        n3473 = local write "Port 1a"(w4538) -> ()
        n3474 = local read "Quit"() -> (w4540:bool)
        n3475 = local write "COM Status"(w4537) -> ()
        n3476 = Select(t=enum16{"init", "MAIN", "Panel Close"}."Panel Close", s=w4540, f=enum16{"init", "MAIN", "Panel Close"}."MAIN") -> (s? t:f=w4539:enum16{"init", "MAIN", "Panel Close"})
      }
      frame "Panel Close" {
      }
      frame Default {
      }
    }
  }
